vi "Joystick and Camera_ms.vi"(10 "VI":bool, 11 "control input":T1) -> (2 "Gantry":dbl[](array[numeric])=[960.6055844814462, 846.5692177804251, 62.66208665532506, 14.77542036630039] format="%#_8g", 3 "control output":T1)   [LabVIEW 2016]
uses:
  Classes/Controller/Camera/Machine Vision.ctl
  Classes/Controller/Controllers.ctl
  Classes/Controller/I-O/I-O.lvclass
  Classes/Controller/Motion/Motion.lvclass
  Classes/Controller/Dispenser/Dispenser.lvclass
  Classes/Controller/Camera/Camera.lvclass
  Classes/Controller/Controller.lvclass
panel:
  in  "Machine Vision 2":T2
  out "Image 2":T3(plugin-control)
  in  "Speed XY":dbl=5.0
  in  "Tab Control":enum32{"jog", "motion"}(tab)=enum."motion"
  in  "Jog Cluster":T4={"Jog XY Cluster"={"object goes up"=FALSE, "object goes down"=FALSE, "object goes right"=FALSE, "object goes left"=FALSE, "SW2"=FALSE, "SW1"=FALSE, "YY (mm)"=0.1, "YN (mm) "=0.01, "NY (mm) "=0.005, "NN (mm) "=0.001}, "Jog Z Cluster "={"Z go down 0.1 mm"=FALSE, "Z go up 0.1 mm"=FALSE, "Z go down 0.05 mm"=FALSE, "Z go up 0.05 mm"=FALSE, "Z go down 0.01 mm"=FALSE, "Z go up 0.01 mm"=FALSE, "Z go down"=FALSE, "Z go up"=FALSE, "step (mm)"=0.001}}
  in  "Lower":bool
  in  "get and go Position":T5={"get P Array"=[FALSE, FALSE, FALSE, FALSE, FALSE], "XY go P Array"=[FALSE, FALSE, FALSE, FALSE, FALSE], "xyzu Position Array"=[[0.0, 0.0, 0.0, 0.0, 0.0], [0.0, 0.0, 0.0, 0.0, 0.0], [0.0, 0.0, 0.0, 0.0, 0.0], [0.0, 0.0, 0.0, 0.0, 0.0]], "XYZ go P Array"=[FALSE, FALSE, FALSE, FALSE, FALSE]}
  in  "Go":bool
  in  "XYZTheta":dbl[](array[numeric])
  in  "Position":dbl
  in  "Z Go":bool
  in  "input position test":dbl[](array[numeric])
  out "XY(F)/XYZ(T)":bool
  out "Array out":dbl[](array[numeric])
  in  "Z Speed":dbl=2.0
  out "Go sum":bool
  in  "Go sum":bool
  in  "light":dbl=5.0
  in  "Change light":bool
  out "XYZTheta Out":dbl[](array[numeric])
  in  "Machine Vision sum":T2
  in  "Record Measurement":bool=TRUE
  in  "Dismount Silicon Tray":bool
  in  "Secure Silicon Tray":bool
  in  "Joystick":bool
  out "Sum":dbl[](array[numeric])
  in  "Stop":bool
  out "Image":T3(plugin-control)
  out "Camera":dbl[](array[numeric])
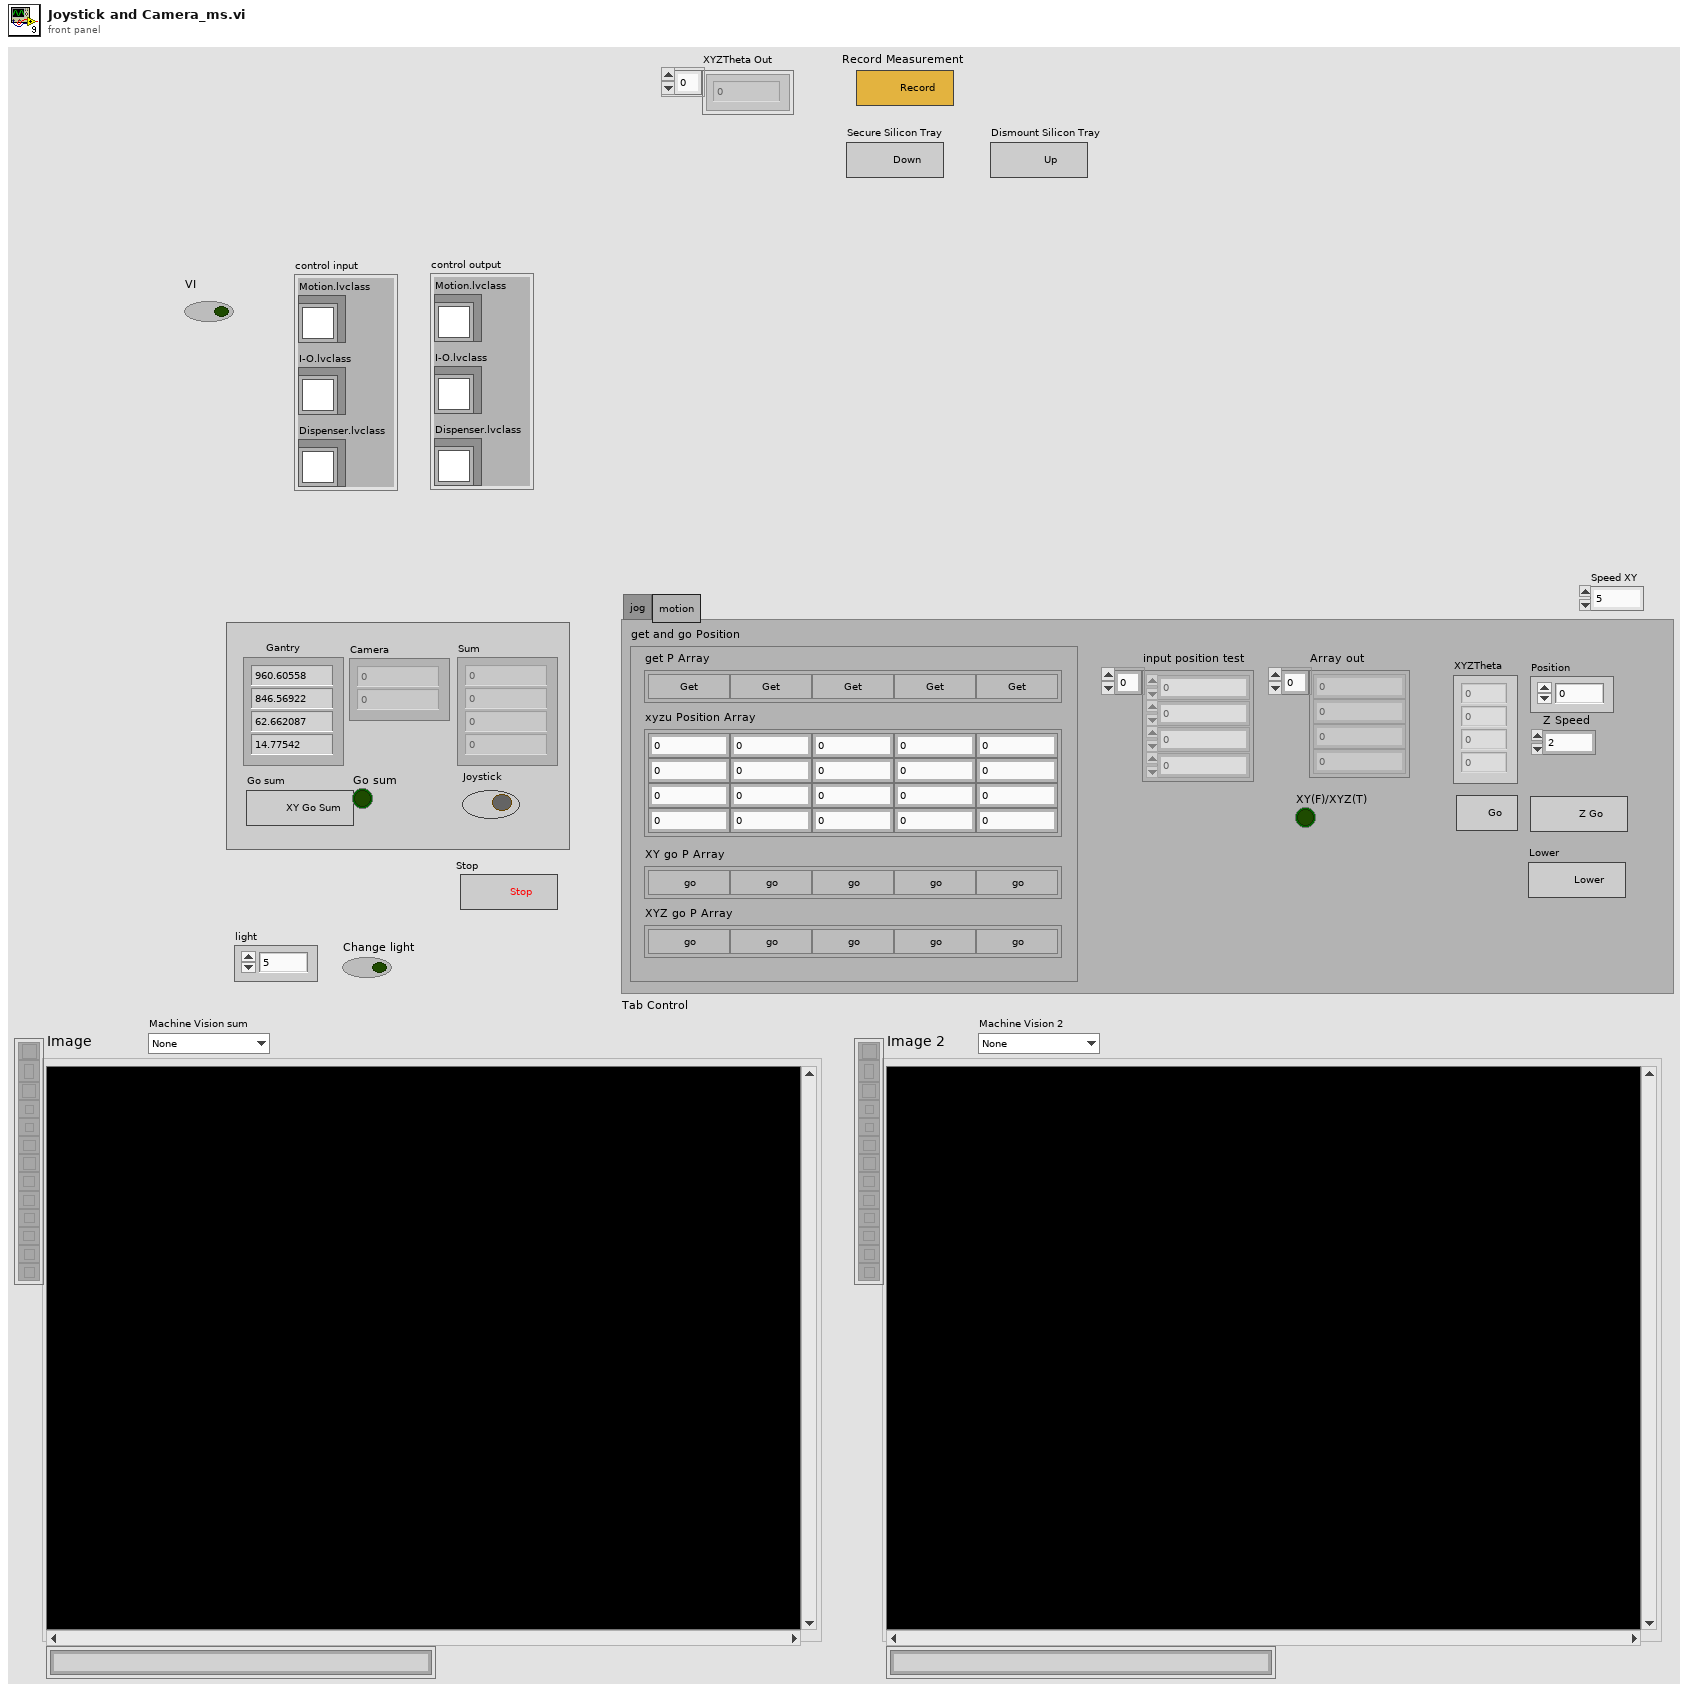
[diagram p1: front panel]
types:
  T1 = typedef "Controller.lvclass/Controllers.ctl" = cluster{"I-O.lvclass":refnum<class "I-O.lvclass">, "Motion.lvclass":refnum<class "Motion.lvclass">, "Dispenser.lvclass":refnum<class "Dispenser.lvclass">}
  T2 = typedef "Camera.lvclass/Machine Vision.ctl" = enum16{"None", "Circle", "Tray Fiducials", "Tray Fiducials, top right", "HPK Silicon square", "HPK Silicon", "8inch PCB Pad", "Hexaboard", "Corner (TL, BR)", "Corner (BL, TR)"}
  T3 = typedef "IMAQ Image.ctl" = refnum<image>
  T4 = cluster{"Jog XY Cluster":cluster{"object goes up":bool, "object goes down":bool, "object goes right":bool, "object goes left":bool, "SW2":bool, "SW1":bool, "YY (mm)":dbl, "YN (mm) ":dbl, "NY (mm) ":dbl, "NN (mm) ":dbl}, "Jog Z Cluster ":cluster{"Z go down 0.1 mm":bool, "Z go up 0.1 mm":bool, "Z go down 0.05 mm":bool, "Z go up 0.05 mm":bool, "Z go down 0.01 mm":bool, "Z go up 0.01 mm":bool, "Z go down":bool, "Z go up":bool, "step (mm)":dbl}}
  T5 = cluster{"get P Array":bool[], "XY go P Array":bool[], "xyzu Position Array":dbl[][], "XYZ go P Array":bool[]}
  T6 = typedef "I-O.lvclass/Pin Map.ctl" = cluster{"Region Valves":i32[], "Extra Valves":dbl[][][], "Tool Primary Valve":i32, "Tool Secondary Valve":i32, "Region Sensors":i32[], "Extra Sensors":dbl[][][], "Tool Primary Sensor":dbl, "Tool Secondary Sensor":dbl, "Compression Sensor":dbl, "5V":i32}
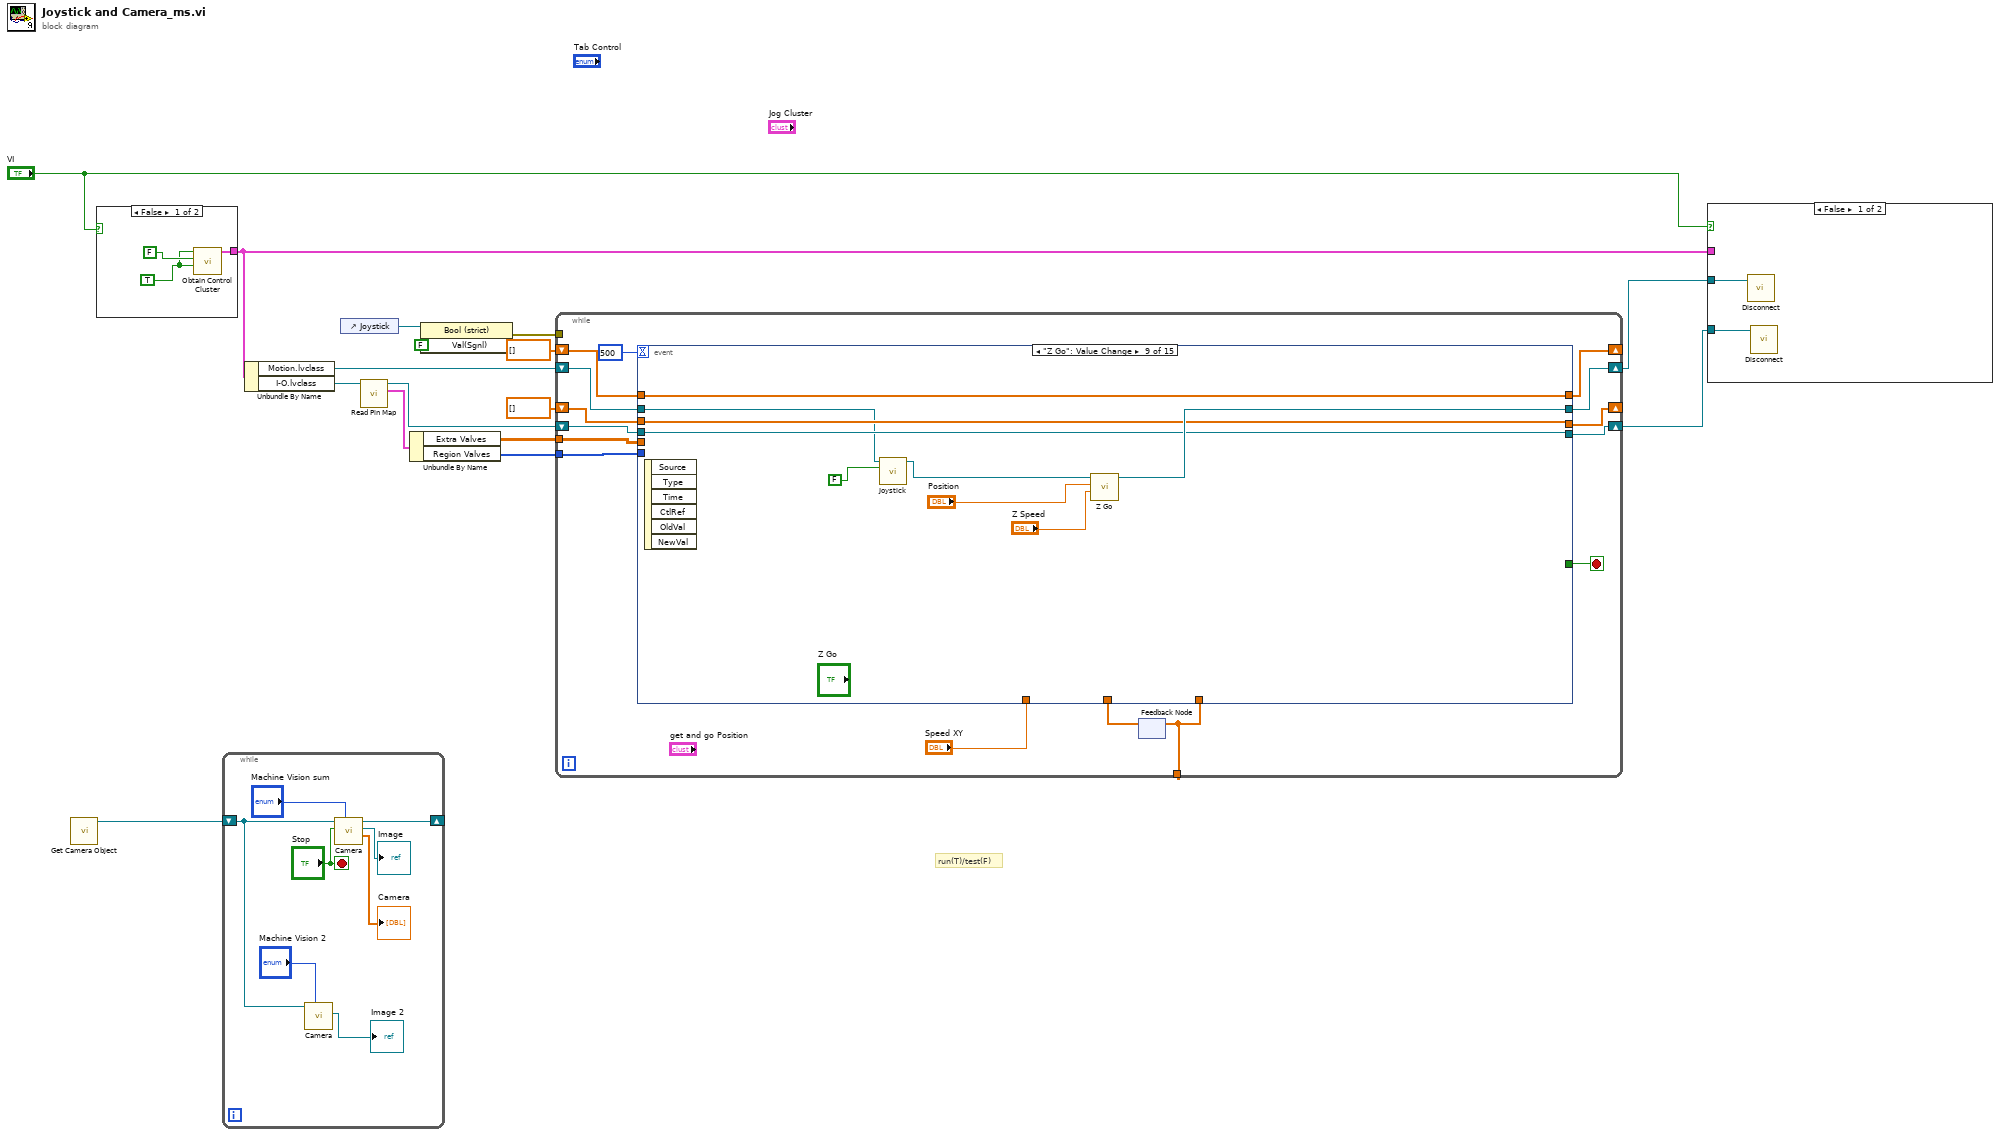
[diagram p0: block diagram]
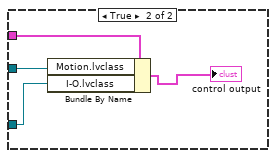
[diagram p2: hidden frame]
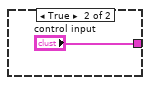
[diagram p3: hidden frame]
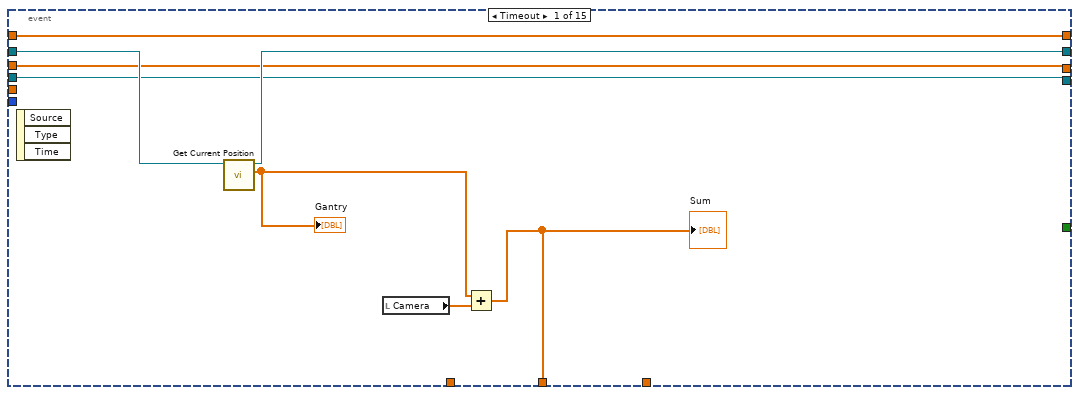
[diagram p4: hidden frame]
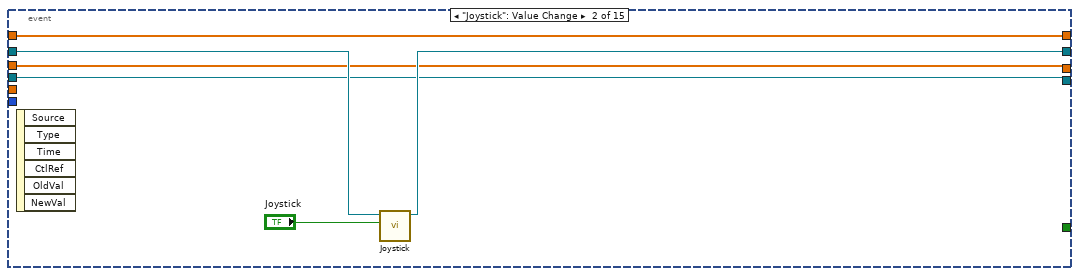
[diagram p5: hidden frame]
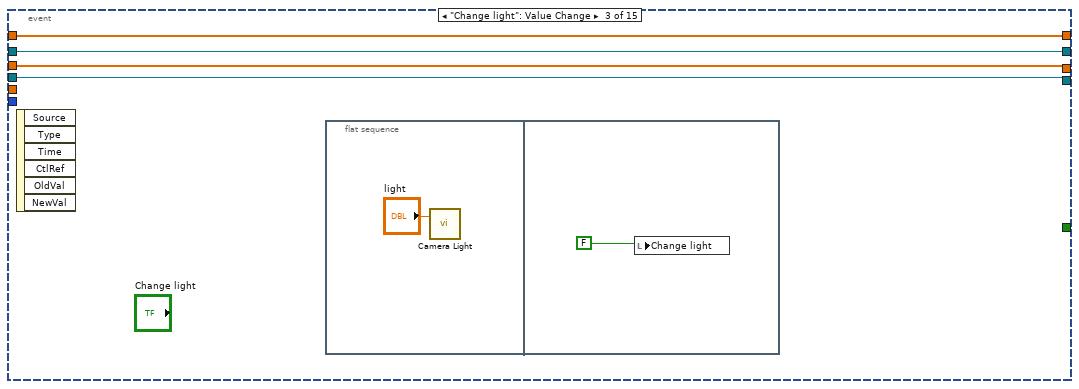
[diagram p6: hidden frame]
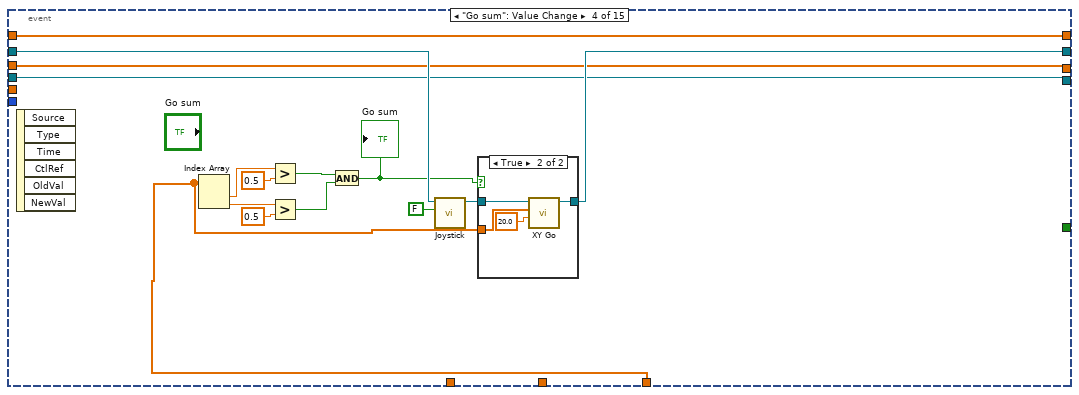
[diagram p7: hidden frame]
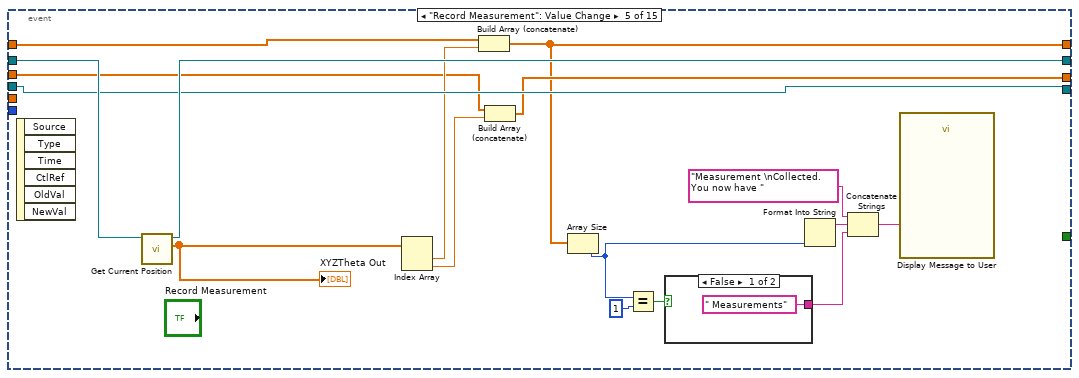
[diagram p9: hidden frame]
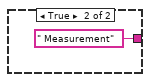
[diagram p10: hidden frame]
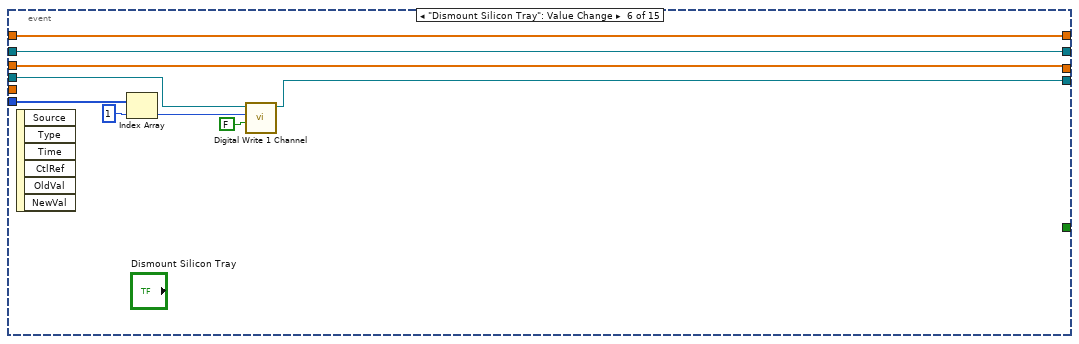
[diagram p11: hidden frame]
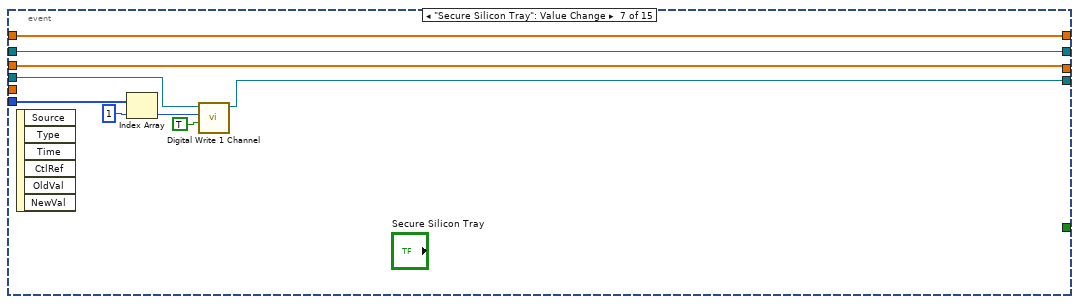
[diagram p12: hidden frame]
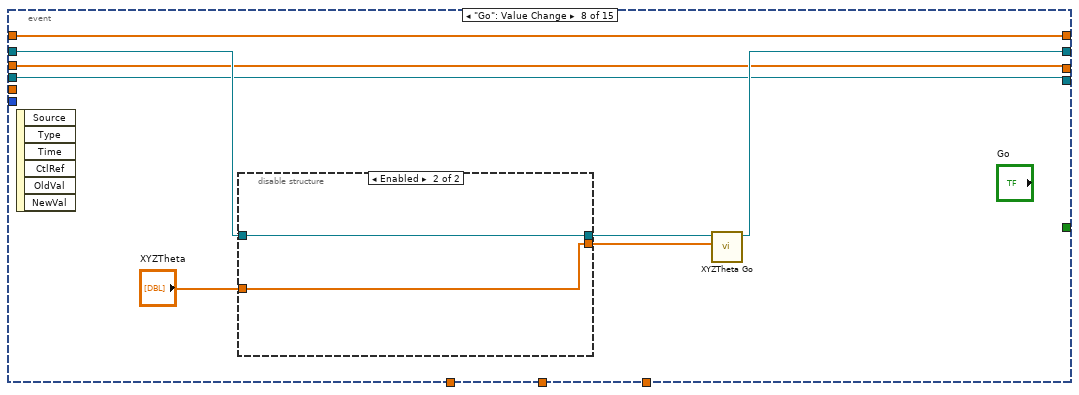
[diagram p13: hidden frame]
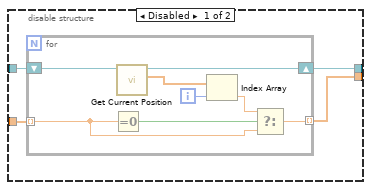
[diagram p14: hidden frame]
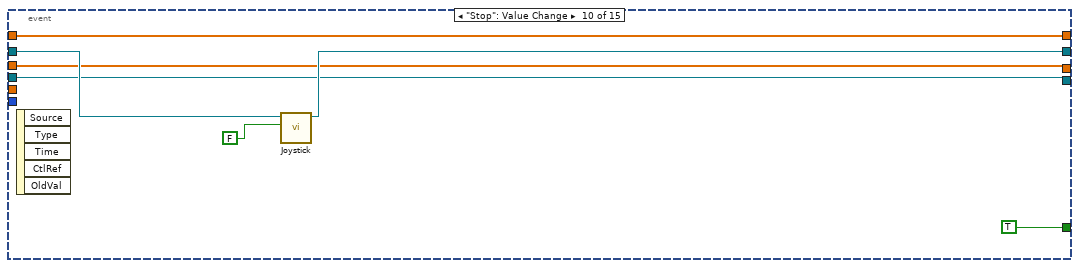
[diagram p15: hidden frame]
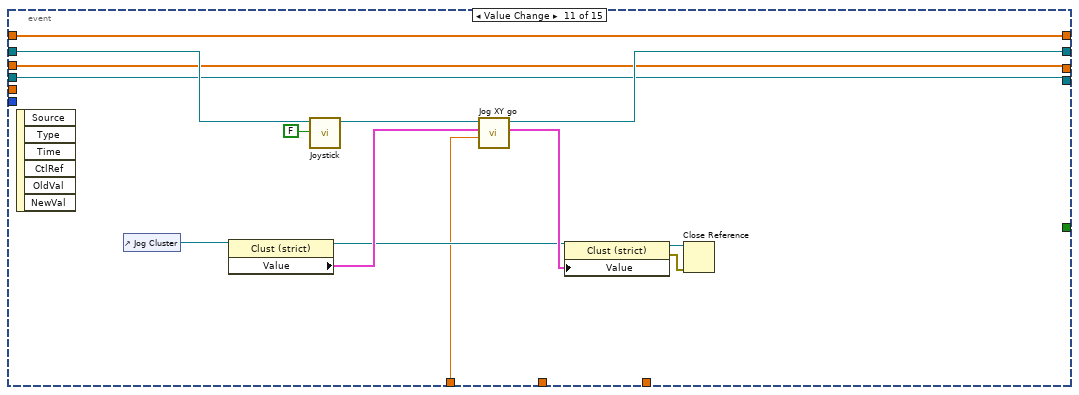
[diagram p16: hidden frame]
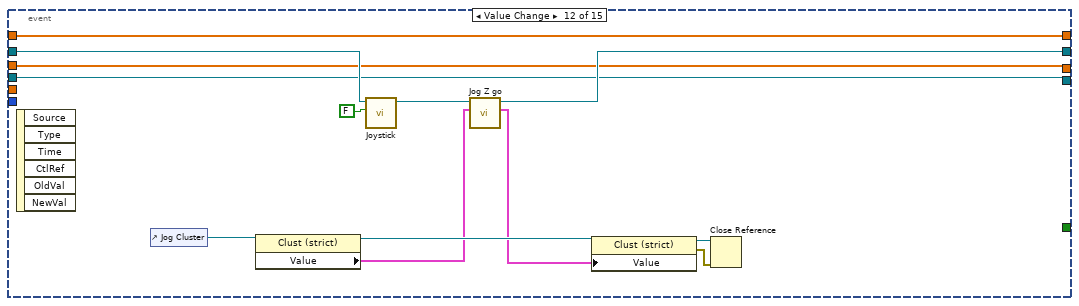
[diagram p17: hidden frame]
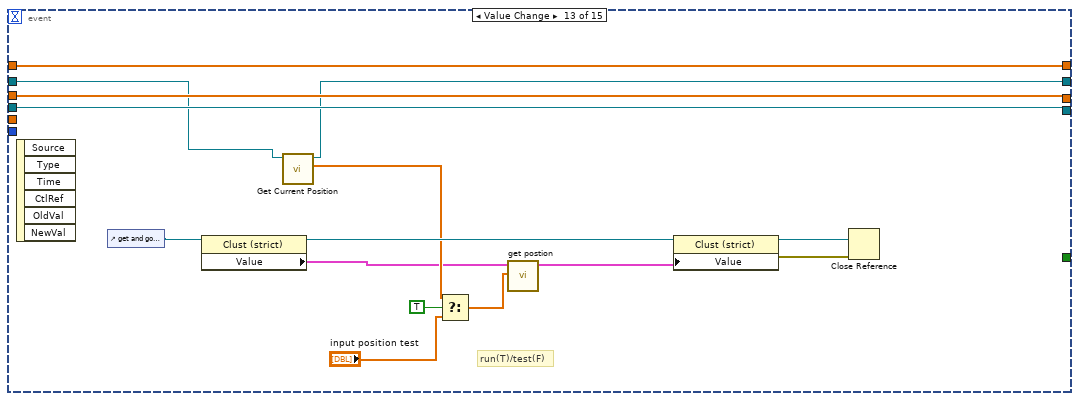
[diagram p18: hidden frame]
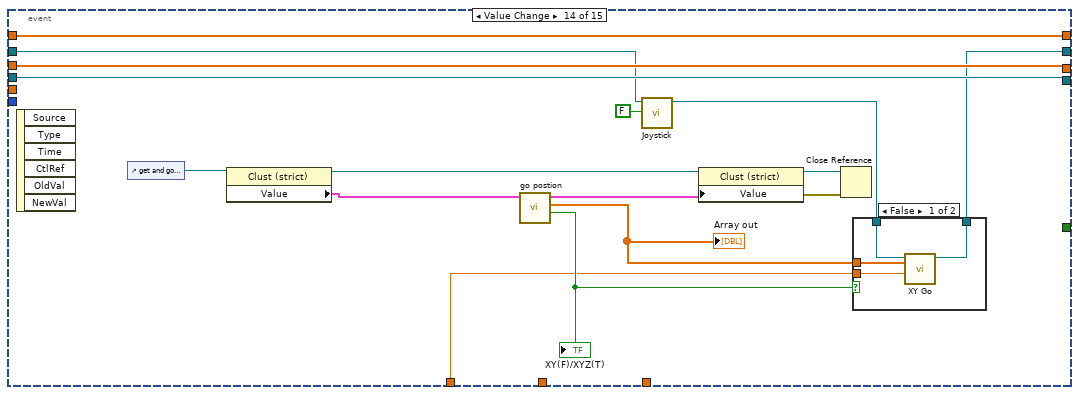
[diagram p19: hidden frame]
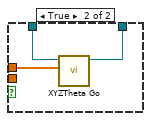
[diagram p20: hidden frame]
diagram:
  # "run(T)/test(F)"
  n1 = call "Get Camera Object.vi"() -> ("Camera out"=w11:refnum<class "Camera.lvclass">)  [unwired: 10 in, 1 out]
  n2 = case shown="False" "VI" {
    tunnel: [w18 "control input"] -> w1
    frame False {
      w17 = TRUE ("I/O")
      n3 = call "Obtain Control Cluster.vi"("I/O"=w17, "Dispense"=FALSE, "Motion"=w17) -> ("Control Out"=w18:T1)  [unwired: 8 in]
    }
    frame True {
    }
  }
  n4 = while {
    shift-right: [w28] -> _
    shift-left: w11 -> [w21]
    stop <- "Stop" stop-if-true
    n5 = call "Camera.vi"("Machine Vision"="Machine Vision 2", "Camera in"=w21) -> ("Image"=→"Image 2":T3)  [unwired: 6 in, 3 out]
    n6 = call "Camera.vi"("Machine Vision"="Machine Vision sum", "Stop"="Stop", "Camera in"=w21) -> ("Camera"=→"Camera":dbl[], "Image"=→"Image":T3, "Camera out"=w28:refnum<class "Camera.lvclass">)  [unwired: 5 in, 1 out]
  }
  n7 = Unbundle By Name(w1) -> ("Motion.lvclass"=w12:refnum<class "Motion.lvclass">, "I-O.lvclass"=w10:refnum<class "I-O.lvclass">)
  n8 = control-ref of="Joystick"() -> (w15:refnum<vi>)
  n9 = call-dynamic "Read Pin Map.vi"("I-O in"=w10) -> ("Pin Map 2"=w8:T6, "I-O out"=w9:refnum<class "I-O.lvclass">)  [unwired: 8 in, 1 out]
  n10 = Unbundle By Name(w8) -> ("Extra Valves"=w6:dbl[][][], "Region Valves"=w7:i32[])
  n11 = property class="Bool (strict)"(reference=w15, "Val(Sgnl)"=FALSE ("Value (Signaling)")) -> (error out=w13:errorcluster)  [unwired: 1 in, 1 out]
  n12 = while {
    shift-right: [w40] -> w14
    shift-left: w12 -> [w41]
    tunnel: w13 -> [_]
    shift-right: [w38] -> w3
    shift-left: w9 -> [w39]
    tunnel: w7 -> [w37]
    tunnel: w6 -> [w36]
    shift-right: [w33] -> _
    shift-left: dbl[] [] -> [w35]
    shift-right: [w32] -> _
    shift-left: dbl[] [] -> [w34]
    tunnel: [w30] -> _
    stop <- w42 stop-if-true
    n13 = feedback #1() -> (w30:dbl[])  [unwired: 1 in]
    n14 = event shown="[8] \"Z Go\": Value Change" {
      selector: _ -> [_ _ _ _ _ _ _ _ _ _ _ _ _ _ _]
      dyn-events: _ -> [_ _ _ _ _ _ _ _ _ _ _ _ _ _ _]
      timeout: 500 -> [_ _ _ _ _ _ _ _ _ _ _ _ _ _ _]
      tunnel: [_ _ _ _ _ _ _ _ _ TRUE _ _ _ _ _] -> w42
      tunnel: w41 -> [w50 w57 w61 w78 w100 w105 w119 w127 w144 w157 w171 w178 w192 w202 w225]
      tunnel: [w49 w55 w61 w76 w99 w105 w119 w124 w151 w155 w169 w176 w191 w210 w228] -> w40
      tunnel: w39 -> [w48 w54 w60 w67 w98 w109 w120 w123 w149 w154 w162 w173 w197 w216 w230]
      tunnel: [w48 w54 w60 w67 w98 w106 w114 w123 w149 w154 w162 w173 w197 w216 w229] -> w38
      tunnel: w37 -> [_ _ _ _ _ w111 w118 _ _ _ _ _ _ _ _]
      tunnel: w36 -> [_ _ _ _ _ _ _ _ _ _ _ _ _ _ _]
      tunnel: w35 -> [w46 w53 w58 w65 w84 w104 w113 w122 w148 w153 w161 w174 w196 w215 w232]
      tunnel: [w46 w53 w58 w65 w88 w104 w113 w122 w148 w153 w161 w174 w196 w215 w232] -> w33
      tunnel: w34 -> [w45 w52 w59 w64 w85 w103 w112 w121 w147 w152 w160 w175 w195 w214 w231]
      tunnel: [w45 w52 w59 w64 w87 w103 w112 w121 w147 w152 w160 w175 w195 w214 w231] -> w32
      tunnel: [w44 _ _ _ _ _ _ _ _ _ _ _ _ _ _] -> w31
      tunnel: w30 -> [_ _ _ w66 _ _ _ _ _ _ _ _ _ _ _]
      tunnel: "Speed XY" -> [_ _ _ _ _ _ _ _ _ _ w159 _ _ w207 _]
      event Timeout {
        n15 = event-data() -> ()  [unwired: 1 in, 3 out]
        n16 = call-dynamic "Get Current Position.vi"("Motion in"=w50) -> ("XYZTheta Out"=w47:dbl[], "Motion out"=w49:refnum<class "Motion.lvclass">)  [unwired: 8 in, 1 out]
        "Gantry" <- w47
        n17 = local read "Camera"() -> (w51:dbl[])
        n18 = Add(x=w47, y=w51) -> (x+y=w44:dbl[])
        "Sum" <- w44
      }
      event "Joystick": Value Change {
        n19 = event-data() -> ()  [unwired: 1 in, 6 out]
        n20 = call-dynamic "Joystick.vi"("Joystick"="Joystick", "Motion in"=w57) -> ("Motion out"=w55:refnum<class "Motion.lvclass">)  [unwired: 8 in, 1 out]
      }
      event "Change light": Value Change {
        n21 = event-data() -> ()  [unwired: 1 in, 6 out]
        n22 = flat-sequence {
          frame #0 {
            n23 = call "Camera Light.vi"("input"="light") -> ()  [unwired: 2 in, 1 out]
          }
          frame #1 {
            n24 = local write "Change light"(FALSE) -> ()
          }
        }
      }
      event "Go sum": Value Change {
        n25 = event-data() -> ()  [unwired: 1 in, 6 out]
        n26 = Index Array(array=w66) -> (element #1=w70:dbl, element #2=w69:dbl)  [unwired: 2 in]
        n27 = Greater?(x=w70, y=0.5) -> (0:w73:bool)
        n28 = Greater?(x=w69, y=0.5) -> (0:w72:bool)
        n29 = And(x=w73, y=w72) -> (x .and. y?=w71:bool)
        "Go sum" <- w71
        n30 = call-dynamic "Joystick.vi"("Joystick"=FALSE, "Motion in"=w78) -> ("Motion out"=w77:refnum<class "Motion.lvclass">)  [unwired: 8 in, 1 out]
        n31 = case shown="True" w71 {
          tunnel: w77 -> [w79 w83]
          tunnel: [w79 w82] -> w76
          tunnel: w66 -> [_ w81]
          frame False {
          }
          frame True {
            n32 = call-dynamic "XY Go.vi"("Speed"=20.0, "XY"=w81, "Motion in"=w83) -> ("Motion out"=w82:refnum<class "Motion.lvclass">)  [unwired: 7 in, 1 out]
          }
        }
      }
      event "Record Measurement": Value Change {
        n33 = event-data() -> ()  [unwired: 1 in, 6 out]
        n34 = call-dynamic "Get Current Position.vi"("Motion in"=w100) -> ("XYZTheta Out"=w89:dbl[], "Motion out"=w99:refnum<class "Motion.lvclass">)  [unwired: 8 in, 1 out]
        "XYZTheta Out" <- w89
        n35 = Index Array(array=w89) -> (element #1=w97:dbl, element #2=w86:dbl)  [unwired: 2 in]
        n36 = Build Array (concatenate) "Build Array"(w85, w97) -> (w87:dbl[])
        n37 = Build Array (concatenate)(w84, w86) -> (w88:dbl[])
        n38 = Array Size(array=w87) -> (size(s)=w92:i32)
        n39 = Equal?(x=w92, y=1) -> (x = y?=w91:bool)
        n40 = case shown="False" w91 {
          tunnel: [" Measurements" " Measurement"] -> w90
          frame False {
          }
          frame True {
          }
        }
        n41 = Format Into String(w92) -> (resulting string=w96:string)  [unwired: 3 in, 1 out]
        n42 = Concatenate Strings("Measurement \nCollected. You now have ", w96, w90) -> (w94:string)
        n43 = call "Display Message to User"("Message"=w94) -> ()  [unwired: 9 in, 2 out]
      }
      event "Dismount Silicon Tray": Value Change {
        n44 = event-data() -> ()  [unwired: 1 in, 6 out]
        n45 = Index Array(array=w111, index=1) -> (element=w108:i32)
        n46 = call-dynamic "Digital Write 1 Channel.vi"("Value"=FALSE, "Channel"=w108, "I-O.lvclass"=w109) -> ("I-O.lvclass 2"=w106:refnum<class "I-O.lvclass">)  [unwired: 7 in, 1 out]
      }
      event "Secure Silicon Tray": Value Change {
        n47 = event-data() -> ()  [unwired: 1 in, 6 out]
        n48 = Index Array(array=w118, index=1) -> (element=w116:i32)
        n49 = call-dynamic "Digital Write 1 Channel.vi"("Value"=TRUE, "Channel"=w116, "I-O.lvclass"=w120) -> ("I-O.lvclass 2"=w114:refnum<class "I-O.lvclass">)  [unwired: 7 in, 1 out]
      }
      event "Go": Value Change {
        n50 = event-data() -> ()  [unwired: 1 in, 6 out]
        n51 = disable-structure shown="Enabled" {
          disable-tunnel: "XYZTheta" -> [w132 w141]
          disable-tunnel: w127 -> [w131 w142]
          disable-tunnel: [w130 w141] -> w126
          disable-tunnel: [w129 w142] -> w125
          frame Disabled {
            n52 = for {
              tunnel: w132 -> [w138] mode=indexing
              tunnel: [w136] -> w130 mode=indexing
              shift-right: [w134] -> w129
              shift-left: w131 -> [w135]
              i -> [w140]
              n53 = Equal To 0?(x=w138) -> (x = 0?=w139:bool)
              n54 = call-dynamic "Get Current Position.vi"("Motion in"=w135) -> ("XYZTheta Out"=w133:dbl[], "Motion out"=w134:refnum<class "Motion.lvclass">)  [unwired: 8 in, 1 out]
              n55 = Index Array(array=w133, index=w140) -> (element=w137:dbl)
              n56 = Select(t=w137, s=w139, f=w138) -> (s? t:f=w136:dbl)
            }
          }
          frame Enabled {
          }
        }
        n57 = call "XYZTheta Go.vi"("XYZTheta In"=w126, "Motion in"=w125) -> ("Motion out"=w124:refnum<class "Motion.lvclass">)  [unwired: 7 in, 2 out]
      }
      event "Z Go": Value Change {
        n58 = event-data() -> ()  [unwired: 1 in, 6 out]
        n59 = call-dynamic "Joystick.vi"("Joystick"=FALSE, "Motion in"=w144) -> ("Motion out"=w143:refnum<class "Motion.lvclass">)  [unwired: 8 in, 1 out]
        n60 = call-dynamic "Z Go.vi"("Speed"="Z Speed", "Position"="Position", "Motion in"=w143) -> ("Motion out"=w151:refnum<class "Motion.lvclass">)  [unwired: 7 in, 1 out]
      }
      event "Stop": Value Change {
        n61 = event-data() -> ()  [unwired: 1 in, 5 out]
        n62 = call-dynamic "Joystick.vi"("Joystick"=FALSE, "Motion in"=w157) -> ("Motion out"=w155:refnum<class "Motion.lvclass">)  [unwired: 8 in, 1 out]
      }
      event "Jog Cluster.Jog XY Cluster.object goes up", "Jog Cluster.Jog XY Cluster.object goes down", "Jog Cluster.Jog XY Cluster.object goes right", "Jog Cluster.Jog XY Cluster.object goes left": Value Change {
        n63 = event-data() -> ()  [unwired: 1 in, 6 out]
        n64 = control-ref of="Jog Cluster"() -> (w168:refnum<vi>)
        n65 = property class="Clust (strict)"(reference=w168) -> (reference out=w165:refnum<vi>, "Value"=w167:T4)  [unwired: 1 in, 1 out]
        n66 = call-dynamic "Joystick.vi"("Joystick"=FALSE, "Motion in"=w171) -> ("Motion out"=w170:refnum<class "Motion.lvclass">)  [unwired: 8 in, 1 out]
        n67 = call "Jog XY go.vi"("Speed"=w159, "Jog Cluster IN"=w167, "Motion.lvclass IN"=w170) -> ("Jog Cluster OUT"=w166:T4, "Motion.lvclass OUT"=w169:refnum<class "Motion.lvclass">)  [unwired: 7 in]
        n68 = property class="Clust (strict)"(reference=w165, "Value"=w166) -> (reference out=w163:refnum<vi>, error out=w164:errorcluster)  [unwired: 1 in]
        n69 = Close Reference(reference=w163, error in (no error)=w164) -> ()  [unwired: 1 out]
      }
      event "Jog Cluster.Jog Z Cluster.Z go down 0.1 mm", "Jog Cluster.Jog Z Cluster.Z go up 0.1 mm", "Jog Cluster.Jog Z Cluster.Z go down 0.05 mm", "Jog Cluster.Jog Z Cluster.Z go up 0.05 mm", "Jog Cluster.Jog Z Cluster.Z go down 0.01 mm", "Jog Cluster.Jog Z Cluster.Z go up 0.01 mm", "Jog Cluster.Jog Z Cluster.Z go down", "Jog Cluster.Jog Z Cluster.Z go up": Value Change {
        n70 = event-data() -> ()  [unwired: 1 in, 6 out]
        n71 = control-ref of="Jog Cluster"() -> (w185:refnum<vi>)
        n72 = property class="Clust (strict)"(reference=w185) -> (reference out=w184:refnum<vi>, "Value"=w181:T4)  [unwired: 1 in, 1 out]
        n73 = call-dynamic "Joystick.vi"("Joystick"=FALSE, "Motion in"=w178) -> ("Motion out"=w177:refnum<class "Motion.lvclass">)  [unwired: 8 in, 1 out]
        n74 = call "Jog Z go.vi"("Jog Cluster IN"=w181, "Motion.lvclass IN"=w177) -> ("Jog Cluster OUT"=w180:T4, "Motion.lvclass OUT"=w176:refnum<class "Motion.lvclass">)  [unwired: 8 in]
        n75 = property class="Clust (strict)"(reference=w184, "Value"=w180) -> (reference out=w182:refnum<vi>, error out=w183:errorcluster)  [unwired: 1 in]
        n76 = Close Reference(reference=w182, error in (no error)=w183) -> ()  [unwired: 1 out]
      }
      event "get and go Position.get P Array": Value Change {
        # "run(T)/test(F)"
        n77 = event-data() -> ()  [unwired: 1 in, 6 out]
        n78 = control-ref of="get and go Position"() -> (w188:refnum<vi>)
        n79 = property class="Clust (strict)"(reference=w188) -> (reference out=w200:refnum<vi>, "Value"=w187:T5)  [unwired: 1 in, 1 out]
        n80 = call-dynamic "Get Current Position.vi"("Motion in"=w192) -> ("XYZTheta Out"=w193:dbl[], "Motion out"=w191:refnum<class "Motion.lvclass">)  [unwired: 8 in, 1 out]
        n81 = Select(t=w193, s=TRUE, f="input position test") -> (s? t:f=w189:dbl[])
        n82 = call "get postion.vi"("Array"=w189, "get and go Position in"=w187) -> ("get and go Position out"=w186:T5)  [unwired: 9 in]
        n83 = property class="Clust (strict)"(reference=w200, "Value"=w186) -> (reference out=w198:refnum<vi>, error out=w199:errorcluster)  [unwired: 1 in]
        n84 = Close Reference(reference=w198, error in (no error)=w199) -> ()  [unwired: 1 out]
      }
      event "get and go Position.XY go P Array", "get and go Position.XYZ go P Array": Value Change {
        n85 = event-data() -> ()  [unwired: 1 in, 6 out]
        n86 = control-ref of="get and go Position"() -> (w206:refnum<vi>)
        n87 = property class="Clust (strict)"(reference=w206) -> (reference out=w213:refnum<vi>, "Value"=w204:T5)  [unwired: 1 in, 1 out]
        n88 = call "go postion.vi"("get and go Position in"=w204) -> ("XY(F)/XYZ(T)"=w209:bool, "Array out"=w208:dbl[], "get and go Position out"=w205:T5)  [unwired: 8 in]
        "Array out" <- w208
        "XY(F)/XYZ(T)" <- w209
        n89 = call-dynamic "Joystick.vi"("Joystick"=FALSE, "Motion in"=w202) -> ("Motion out"=w201:refnum<class "Motion.lvclass">)  [unwired: 8 in, 1 out]
        n90 = property class="Clust (strict)"(reference=w213, "Value"=w205) -> (reference out=w211:refnum<vi>, error out=w212:errorcluster)  [unwired: 1 in]
        n91 = Close Reference(reference=w211, error in (no error)=w212) -> ()  [unwired: 1 out]
        n92 = case shown="False" w209 {
          tunnel: w201 -> [w220 w223]
          tunnel: [w219 w222] -> w210
          tunnel: w208 -> [w218 w221]
          tunnel: w207 -> [w217 _]
          frame False {
            n93 = call-dynamic "XY Go.vi"("Speed"=w217, "XY"=w218, "Motion in"=w220) -> ("Motion out"=w219:refnum<class "Motion.lvclass">)  [unwired: 7 in, 1 out]
          }
          frame True {
            n94 = call "XYZTheta Go.vi"("XYZTheta In"=w221, "Motion in"=w223) -> ("Motion out"=w222:refnum<class "Motion.lvclass">)  [unwired: 7 in, 2 out]
          }
        }
      }
      event "Lower": Value Change {
        n95 = event-data() -> ()  [unwired: 1 in, 6 out]
        n96 = call-dynamic "Joystick.vi"("Joystick"=FALSE, "Motion in"=w225) -> ("Motion out"=w224:refnum<class "Motion.lvclass">)  [unwired: 8 in, 1 out]
        n97 = call "Lower stop.vi"("Motion.lvclass 2"=w224, "I-O.lvclass"=w230) -> ("error out"=w227:errorcluster, "Motion.lvclass"=w228:refnum<class "Motion.lvclass">, "I-O out"=w229:refnum<class "I-O.lvclass">)  [unwired: 7 in]
        n98 = flat-sequence {
          tunnel: w227 -> [_]
          frame #0 {
            n99 = control-ref of="Lower"() -> (w234:refnum<vi>)
            n100 = property class="Bool (strict)"(reference=w234, "Value"=FALSE) -> (reference out=w235:refnum<vi>, error out=w236:errorcluster)  [unwired: 1 in]
            n101 = Close Reference(reference=w235, error in (no error)=w236) -> ()  [unwired: 1 out]
          }
        }
      }
    }
    n102 = feedback-in #1(w31) -> ()
  }
  n103 = case shown="False" "VI" {
    tunnel: w14 -> [w238 w240]
    tunnel: w3 -> [w237 w241]
    tunnel: w1 -> [_ w242]
    frame False {
      n104 = call-dynamic "Disconnect.vi"("Controller in"=w238) -> ()  [unwired: 9 in, 1 out]
      n105 = call-dynamic "Disconnect.vi"("I-O in"=w237) -> ()  [unwired: 9 in, 1 out]
    }
    frame True {
      n106 = Bundle By Name(cluster=w242, "Motion.lvclass"=w240, "I-O.lvclass"=w241) -> (→"control output":T1)
    }
  }
